vi "Draw Water And Sky.vi"(10 "Pixel Data in":u32[][](array[numeric]), 11 "Rotating Objects in":refnum<class "Rotating Objects.lvclass">) -> (2 "Pixel Data out":u32[][](array[numeric]), 3 "Rotating Objects out":refnum<class "Rotating Objects.lvclass">)   [LabVIEW 2020, in "Amnesia.lvlib" / "Rotating Objects.lvclass"]
uses:
  Rotating Objects.lvclass
  <vilib>/Analysis/NI_AALBase.lvlib
  <vilib>/Analysis/1siggen.llb/Ramp Pattern by Samples.vi
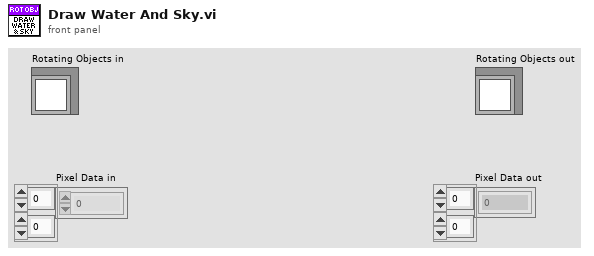
[diagram p1: front panel]
types:
  T1 = typedef "Raster.lvlib/Rectangle Dimensions.ctl" = cluster{"Width":u32, "Height":u32}
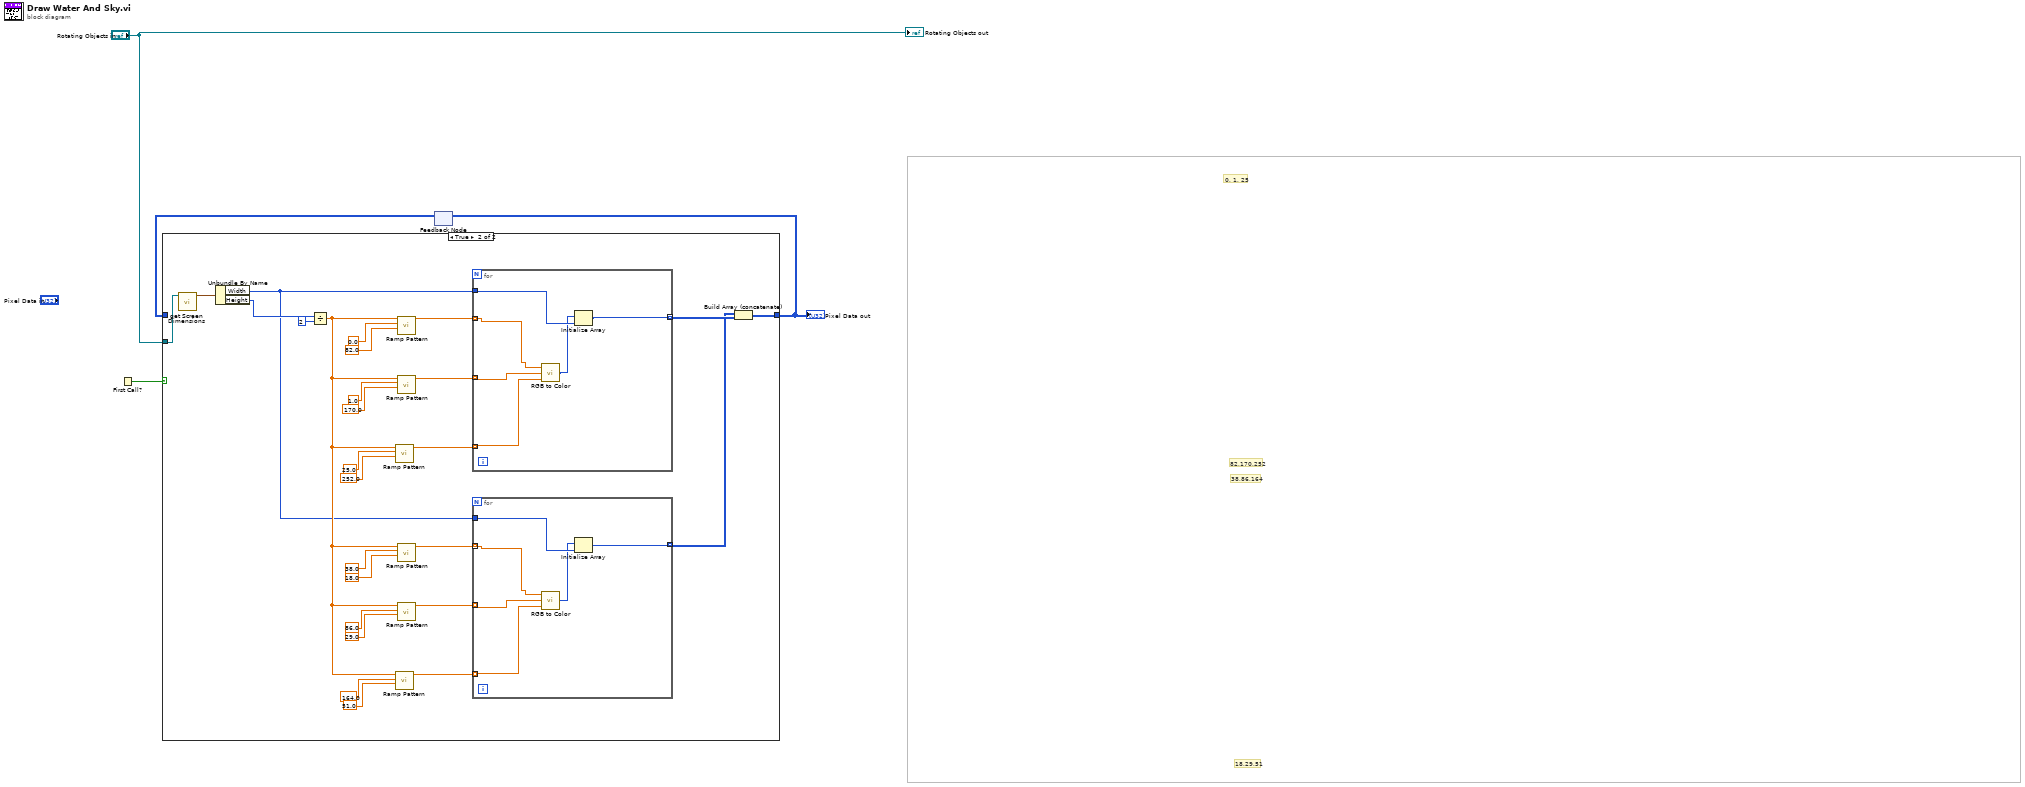
[diagram p0: block diagram]
diagram:
  # "18,29,51"
  # "38,86,164"
  # "82,170,252"
  # "0, 1, 25"
  n1 = First Call?() -> (First Call?: T/F=w1:bool)
  n2 = feedback #1() -> (w2:u32[][])  [unwired: 1 in]
  n3 = case shown="True" w1 {
    tunnel: "Rotating Objects in" -> [_ w32]
    tunnel: [w5 w8] -> w3
    tunnel: w2 -> [w5 _]
    frame False {
    }
    frame True {
      n4 = call-dynamic "get Screen Dimensions.vi"("Scene in"=w32) -> ("Rectangle Dimensions"=w31:T1)  [unwired: 10 in]
      n5 = Unbundle By Name(w31) -> ("Width"=w6:u32, "Height"=w30:u32)
      n6 = Divide(x=w30, y=u32 2) -> (x/y=w7:dbl)
      n7 = call-poly <vilib>:"Ramp Pattern.vi"("start"=252.0, "end"=25.0, "samples"=w7) -> ("Ramp Pattern"=w20:dbl[])  [unwired: 7 in, 1 out]
      n8 = call-poly <vilib>:"Ramp Pattern.vi"("start"=51.0, "end"=164.0, "samples"=w7) -> ("Ramp Pattern"=w19:dbl[])  [unwired: 7 in, 1 out]
      n9 = call-poly <vilib>:"Ramp Pattern.vi"("start"=82.0, "end"=0.0, "samples"=w7) -> ("Ramp Pattern"=w22:dbl[])  [unwired: 7 in, 1 out]
      n10 = call-poly <vilib>:"Ramp Pattern.vi"("start"=170.0, "end"=1.0, "samples"=w7) -> ("Ramp Pattern"=w21:dbl[])  [unwired: 7 in, 1 out]
      n11 = call-poly <vilib>:"Ramp Pattern.vi"("start"=18.0, "end"=38.0, "samples"=w7) -> ("Ramp Pattern"=w17:dbl[])  [unwired: 7 in, 1 out]
      n12 = call-poly <vilib>:"Ramp Pattern.vi"("start"=29.0, "end"=86.0, "samples"=w7) -> ("Ramp Pattern"=w18:dbl[])  [unwired: 7 in, 1 out]
      n13 = for {
        tunnel: w22 -> [w43] mode=indexing
        tunnel: w21 -> [w42] mode=indexing
        tunnel: w20 -> [w41] mode=indexing
        tunnel: w6 -> [w44]
        tunnel: [w39] -> w10 mode=indexing
        n14 = call <vilib>:"RGB to Color.vi"("B"=w41, "G"=w42, "R"=w43) -> ("Color"=w40:u32)
        n15 = Initialize Array(w40, w44) -> (w39:u32[])
      }
      n16 = for {
        tunnel: w17 -> [w37] mode=indexing
        tunnel: w18 -> [w36] mode=indexing
        tunnel: w19 -> [w35] mode=indexing
        tunnel: w6 -> [w38]
        tunnel: [w33] -> w9 mode=indexing
        n17 = call <vilib>:"RGB to Color.vi"("B"=w35, "G"=w36, "R"=w37) -> ("Color"=w34:u32)
        n18 = Initialize Array(w34, w38) -> (w33:u32[])
      }
      n19 = Build Array (concatenate)(w9, w10) -> (w8:u32[][])
    }
  }
  "Pixel Data out" <- w3
  n20 = feedback-in #1(w3) -> ()
  "Rotating Objects out" <- "Rotating Objects in"
